vi "UHR-Fleezers Control (host) - 12.0(oscillate_test).vi"() -> ()   [LabVIEW 2014] (continued)
            n2102 = Wait (ms)(milliseconds to wait=u32 250) -> ()  [unwired: 1 out]
          }
          frame #5 {
            n2103 = case shown="\"1\"" "Remove Action Offset Dropdown" {
              tunnel: TRUE ("Value (Signaling)") -> [w3014 w3022 w3030]
              frame "1" {
                n2104 = flat-sequence {
                  tunnel: w3014 -> [w3021]
                  frame #0 {
                    n2105 = local read "factor"() -> (w3016:dbl)
                    n2106 = Greater Than 0?(x=w3016) -> (x > 0?=w3020:bool)
                    n2107 = Select(t=1.0, s=w3020, f=-1.0) -> (s? t:f=w3017:dbl)
                    n2108 = Multiply(x=w3017, y=w3016) -> (x*y=w3015:dbl)
                    n2109 = local write "factor"(w3015) -> ()
                  }
                  frame #1 {
                    n2110 = property on="Remove Offset to factor" class="Bool (strict)"("Val(Sgnl)"=w3021) -> ()  [unwired: 2 in, 2 out]
                  }
                }
              }
              frame "2" {
                n2111 = flat-sequence {
                  tunnel: w3022 -> [w3029]
                  frame #0 {
                    n2112 = local read "factor"() -> (w3023:dbl)
                    n2113 = Greater Than 0?(x=w3023) -> (x > 0?=w3028:bool)
                    n2114 = Select(t=-1.0, s=w3028, f=1.0) -> (s? t:f=w3026:dbl)
                    n2115 = Multiply(x=w3023, y=w3026) -> (x*y=w3025:dbl)
                    n2116 = local write "factor"(w3025) -> ()
                  }
                  frame #1 {
                    n2117 = property on="Remove Offset to factor" class="Bool (strict)"("Val(Sgnl)"=w3029) -> ()  [unwired: 2 in, 2 out]
                  }
                }
              }
              frame "0", Default {
                n2118 = property on="Remove Action Offset" class="Bool (strict)"("Val(Sgnl)"=w3030) -> ()  [unwired: 2 in, 2 out]
              }
            }
            n2119 = case shown="False" "Trap Trig Fl." {
              frame False {
                n2120 = case shown="True" "Green ON after FB ON?" {
                  selector: "Green ON after FB ON?" -> [_ w3032]
                  frame False {
                  }
                  frame True {
                    n2121 = property on="Green ON/Interlacing" class="Bool (strict)"("Val(Sgnl)"=w3032) -> ()  [unwired: 2 in, 2 out]
                  }
                }
              }
              frame True {
              }
            }
            n2122 = Wait (ms)(milliseconds to wait=u32 250) -> ()  [unwired: 1 out]
          }
          frame #6 {
            n2123 = property on="Start Saving" class="Bool (strict)"("Val(Sgnl)"=TRUE ("Value (Signaling)")) -> ()  [unwired: 2 in, 2 out]
            n2124 = Wait (ms)(milliseconds to wait=u32 5000) -> ()  [unwired: 1 out]
          }
          frame #7 {
            w3036 = TRUE ("Value (Signaling)")
            n2125 = property on="Rem fb disp offset" class="Bool (strict)"("Val(Sgnl)"=w3036) -> ()  [unwired: 2 in, 2 out]
            n2126 = property on="Remove Offset" class="Bool (strict)"("Val(Sgnl)"=w3036) -> ()  [unwired: 2 in, 2 out]
            n2127 = Wait (ms)(milliseconds to wait=u32 100) -> ()  [unwired: 1 out]
          }
          frame #8 {
            n2128 = case shown="True" w3039 {
              frame False {
              }
              frame True {
                n2129 = local write "Trap Trig. Fl."(TRUE ("Value (Signaling)")) -> ()
              }
            }
          }
          frame #9 {
            n2130 = local read "Tether"() -> (w3042:bool)
            n2131 = And(x="Start dipping after?", y=w3042) -> (x .and. y?=w3041:bool)
            n2132 = case shown="True" w3041 {
              frame False {
              }
              frame True {
                n2133 = flat-sequence {
                  frame #0 {
                    n2134 = Multiply(x="Delay before dipping (s)", y=1000.0) -> (x*y=w3045:dbl)
                    n2135 = Wait (ms)(milliseconds to wait=w3045) -> ()  [unwired: 1 out]
                  }
                  frame #1 {
                    n2136 = property on="Dip for Protein" class="Bool (strict)"("Val(Sgnl)"=TRUE ("Value (Signaling)")) -> ()  [unwired: 2 in, 2 out]
                    n2137 = local write "Scripts"(T35."Dipping") -> ()
                  }
                }
              }
            }
          }
        }
      }
      event "Rupture Script": Value Change {
        n2138 = event-data() -> ()  [unwired: 1 in, 5 out]
        n2139 = local write "Rupture Script"(FALSE ("Rupture Script")) -> ()
        n2140 = flat-sequence {
          frame #0 {
            w3051 = TRUE
            w3056 = FALSE
            # "Number 6 for now is the\nrupture-experiment\nparameters."
            n2141 = local read "Starting Trap D (MHz)"() -> (w3057:dbl)
            n2142 = local write "Restart DMA? (AOD)"(w3056) -> ()
            n2143 = Replace Array Subset(array=u32[] [0] ("Index Values"), new element=6, index=0) -> (w3052:u32[])
            n2144 = local write "Save scans"(w3056) -> ()
            n2145 = property on="Trap D (MHz)" class="DigNum (strict)"("Val(Sgnl)"=w3057) -> ()  [unwired: 2 in, 2 out]
            n2146 = property on="Saved AOD Raster Scan Parameter Sets" class="Arr (strict)"("Index Values"=w3052) -> ()  [unwired: 2 in, 2 out]
            n2147 = property on="Start Saving" class="Bool (strict)"("Val(Sgnl)"=w3051) -> ()  [unwired: 2 in, 2 out]
            n2148 = property on="Green ON/Interlacing" class="Bool (strict)"("Val(Sgnl)"=w3051) -> ()  [unwired: 2 in, 2 out]
          }
          frame #1 {
            n2149 = property on="Load parameters" class="Bool (strict)"("Val(Sgnl)"=TRUE ("Value (Signaling)")) -> ()  [unwired: 2 in, 2 out]
          }
        }
      }
      event "Fixed Traps Script": Value Change {
        n2150 = event-data() -> ()  [unwired: 1 in, 5 out]
        n2151 = local write "Fixed Traps Script"(FALSE ("Fixed Traps Data\nScript")) -> ()
        n2152 = flat-sequence {
          frame #0 {
            n2153 = case shown="True" "Green ON" {
              frame False {
              }
              frame True {
                n2154 = property on="Green ON/Interlacing" class="Bool (strict)"("Val(Sgnl)"=TRUE) -> ()  [unwired: 2 in, 2 out]
              }
            }
            n2155 = local write "Offset (nm)"(0.0 ("Offset (nm)")) -> ()
            n2156 = property on="Sample Channel\nFlow" class="Bool (strict)"("Val(Sgnl)"=FALSE ("Value (Signaling)")) -> ()  [unwired: 2 in, 2 out]
            n2157 = property on="Trap D (MHz)" class="DigNum (strict)"("Val(Sgnl)"="Fixed Traps Trap Delta (MHz)") -> ()  [unwired: 2 in, 2 out]
          }
          frame #1 {
            n2158 = Wait (ms)(milliseconds to wait=u32 1000) -> ()  [unwired: 1 out]
          }
          frame #2 {
            n2159 = local write "Start Saving"(TRUE ("Start Saving")) -> ()
          }
          frame #3 {
            n2160 = local read "Bead Sep. Int. Time (s)"() -> (w3067:dbl)
            n2161 = Multiply(x=w3067, y=1000.0) -> (x*y=w3069:dbl)
            n2162 = Wait (ms)(milliseconds to wait=w3069) -> ()  [unwired: 1 out]
          }
          frame #4 {
            n2163 = property on="Remove Offset" class="Bool (strict)"("Val(Sgnl)"=TRUE ("Value (Signaling)")) -> ()  [unwired: 2 in, 2 out]
          }
          frame #5 {
            n2164 = property on="Dip for Protein" class="Bool (strict)"("Val(Sgnl)"="Start dipping after?") -> ()  [unwired: 2 in, 2 out]
          }
        }
      }
      event "Got DNA bead": Value Change {
        n2165 = event-data() -> ()  [unwired: 1 in, 5 out]
        n2166 = flat-sequence {
          frame #0 {
            w3073 = FALSE ("Key Focus")
            n2167 = local read "Daq spot flow on"() -> (w3074:bool)
            n2168 = case shown="True" w3074 {
              frame False {
              }
              frame True {
                n2169 = property on="Sample Channel\nFlow" class="Bool (strict)"("Val(Sgnl)"=TRUE ("Value (Signaling)")) -> ()  [unwired: 2 in, 2 out]
              }
            }
            n2170 = local write "Got DNA bead"(w3073) -> ()
            n2171 = property on="Got DNA bead" class="Bool (strict)"("Key Focus"=w3073) -> ()  [unwired: 2 in, 2 out]
          }
          frame #1 {
            n2172 = property on="Inject Pump 1" class="Bool (strict)"("Val(Sgnl)"=FALSE ("Value (Signaling)")) -> ()  [unwired: 2 in, 2 out]
          }
          frame #2 {
            n2173 = property on="Cal/Data Acq. Spot" class="Bool (strict)"("Val(Sgnl)"=TRUE ("Value (Signaling)")) -> ()  [unwired: 2 in, 2 out]
          }
        }
      }
      event "Take Stepping Data": Value Change {
        n2174 = event-data() -> ()  [unwired: 1 in, 5 out]
        n2175 = local read "Save ave N"() -> (w3086:dbl)
        n2176 = flat-sequence {
          tunnel: w3086 -> [w3088]
          tunnel: [w3088] -> w3081
          tunnel: [w3090] -> w3082
          tunnel: w3081 -> [w3090]
          tunnel: [w3092] -> w3083
          tunnel: w3082 -> [w3092]
          tunnel: [w3095] -> w3084
          tunnel: w3083 -> [w3095]
          tunnel: [w3097] -> w3085
          tunnel: w3084 -> [w3097]
          tunnel: [w3099] -> w3079
          tunnel: w3085 -> [w3099]
          tunnel: w3079 -> [w3102]
          tunnel: [w3102] -> w3078
          tunnel: w3078 -> [w3103]
          tunnel: [w3103] -> w3080
          tunnel: w3080 -> [w3109]
          frame #0 {
            n2177 = property on="Save ave N" class="DigNum (strict)"("Val(Sgnl)"="Save ave factor") -> ()  [unwired: 2 in, 2 out]
          }
          frame #1 {
            n2178 = Wait (ms)(milliseconds to wait=u32 100) -> ()  [unwired: 1 out]
          }
          frame #2 {
            n2179 = local read "Offset 2 Start (MHz)"() -> (w3094:dbl)
            n2180 = property on="Saved AOD Raster Scan Parameter Sets" class="Arr (strict)"("Index Values"=u32[] [2]) -> ()  [unwired: 2 in, 2 out]
            n2181 = property on="Trap D (MHz)" class="DigNum (strict)"("Val(Sgnl)"=w3094) -> ()  [unwired: 2 in, 2 out]
          }
          frame #3 {
            n2182 = property on="Load parameters" class="Bool (strict)"("Val(Sgnl)"=TRUE ("Value (Signaling)")) -> ()  [unwired: 2 in, 2 out]
          }
          frame #4 {
            n2183 = Wait (ms)(milliseconds to wait=u32 100) -> ()  [unwired: 1 out]
          }
          frame #5 {
            n2184 = property on="Trap Raster Scan" class="Bool (strict)"("Val(Sgnl)"=TRUE ("Value (Signaling)")) -> ()  [unwired: 2 in, 2 out]
          }
          frame #6 {
            n2185 = Wait (ms)(milliseconds to wait=u32 1000) -> ()  [unwired: 1 out]
          }
          frame #7 {
            n2186 = while {
              stop <- w3106 stop-if-true
              n2187 = local read "Raster Scanning..."() -> (w3108:bool)
              n2188 = local read "Saving..."() -> (w3107:bool)
              n2189 = Not(x=w3107) -> (.not. x?=w3104:bool)
              n2190 = Not(x=w3108) -> (.not. x?=w3105:bool)
              n2191 = And(x=w3105, y=w3104) -> (x .and. y?=w3106:bool)
            }
          }
          frame #8 {
            n2192 = property on="Save ave N" class="DigNum (strict)"("Val(Sgnl)"=w3109) -> ()  [unwired: 2 in, 2 out]
          }
        }
      }
      event "Step Size (nm)": Value Change {
        n2193 = event-data() -> ()  [unwired: 1 in, 5 out]
        n2194 = flat-sequence {
          frame #0 {
            n2195 = property on="Saved AOD Raster Scan Parameter Sets" class="Arr (strict)"("Index Values"=u32[] [1]) -> ()  [unwired: 2 in, 2 out]
          }
          frame #1 {
            n2196 = Multiply(x="N Steps", y="Step Size (nm)") -> (x*y=w3111:dbl)
            n2197 = property on="Scan Speed AOD (nm/s) 2" class="DigNum (strict)"("Value"="Step Size (nm)") -> ()  [unwired: 2 in, 2 out]
            n2198 = property on="Step Size AOD (nm) 2" class="DigNum (strict)"("Value"="Step Size (nm)") -> ()  [unwired: 2 in, 2 out]
            n2199 = property on="Scan Range AOD (nm) 2" class="DigNum (strict)"("Value"=w3111) -> ()  [unwired: 2 in, 2 out]
          }
        }
      }
      event "Take Detection Laser\nImage": Value Change {
        n2200 = event-data() -> ()  [unwired: 1 in, 5 out]
        n2201 = flat-sequence {
          tunnel: [w3139] -> w3129
          tunnel: [w3138] -> w3122
          tunnel: [w3137] -> w3114
          tunnel: [w3142] -> w3130
          tunnel: w3129 -> [w3142]
          tunnel: [w3141] -> w3123
          tunnel: w3122 -> [w3141]
          tunnel: [w3140] -> w3115
          tunnel: w3114 -> [w3140]
          tunnel: [w3146] -> w3131
          tunnel: w3130 -> [w3146]
          tunnel: [w3145] -> w3124
          tunnel: w3123 -> [w3145]
          tunnel: [w3144] -> w3116
          tunnel: w3115 -> [w3144]
          tunnel: [w3152] -> w3132
          tunnel: w3131 -> [w3152]
          tunnel: [w3151] -> w3125
          tunnel: w3124 -> [w3151]
          tunnel: [w3150] -> w3117
          tunnel: w3116 -> [w3150]
          tunnel: [w3156] -> w3133
          tunnel: w3132 -> [w3156]
          tunnel: [w3155] -> w3126
          tunnel: w3125 -> [w3155]
          tunnel: [w3154] -> w3118
          tunnel: w3117 -> [w3154]
          tunnel: [w3160] -> w3134
          tunnel: w3133 -> [w3160]
          tunnel: [w3159] -> w3127
          tunnel: w3126 -> [w3159]
          tunnel: [w3158] -> w3119
          tunnel: w3118 -> [w3158]
          tunnel: [w3164] -> w3135
          tunnel: w3134 -> [w3164]
          tunnel: [w3163] -> w3128
          tunnel: w3127 -> [w3163]
          tunnel: [w3162] -> w3120
          tunnel: w3119 -> [w3162]
          tunnel: w3135 -> [w3170]
          tunnel: w3128 -> [w3169]
          tunnel: [w3167] -> w3121
          tunnel: w3120 -> [w3167]
          tunnel: w3121 -> [w3171]
          frame #0 {
            n2202 = local read "Laser interlacing mode (all lasers)"() -> (w3138:enum32{"Laser ON", "Laser OFF", "Interlace"})
            n2203 = local read "Green ON/Interlacing"() -> (w3139:bool)
            n2204 = local read "Green FB On/Off"() -> (w3137:bool)
          }
          frame #1 {
            n2205 = property on="Green FB On/Off" class="Bool (strict)"("Val(Sgnl)"=FALSE ("Value (Signaling)")) -> ()  [unwired: 2 in, 2 out]
          }
          frame #2 {
            n2206 = property on="Green ON/Interlacing" class="Bool (strict)"("Val(Sgnl)"=TRUE ("Value (Signaling)")) -> ()  [unwired: 2 in, 2 out]
            n2207 = property on="Flip Green Filter" class="Bool (strict)"("Val(Sgnl)"=TRUE ("Value (Signaling)")) -> ()  [unwired: 2 in, 2 out]
            n2208 = property on="Laser interlacing mode (all lasers)" class="RadioBtnsControl (strict)"("Val(Sgnl)"=enum32{"Laser ON", "Laser OFF", "Interlace"}."Laser ON" ("Value (Signaling)")) -> ()  [unwired: 2 in, 2 out]
          }
          frame #3 {
            n2209 = Wait (ms)(milliseconds to wait=u32 500) -> ()  [unwired: 1 out]
          }
          frame #4 {
            n2210 = property on="Confocal\nImage" class="Bool (strict)"("Val(Sgnl)"=TRUE ("Value (Signaling)")) -> ()  [unwired: 2 in, 2 out]
          }
          frame #5 {
            n2211 = Wait (ms)(milliseconds to wait=u32 2000) -> ()  [unwired: 1 out]
          }
          frame #6 {
            n2212 = while {
              stop <- w3165 stop-if-true
              n2213 = local read "Saving..."() -> (w3166:bool)
              n2214 = Not(x=w3166) -> (.not. x?=w3165:bool)
            }
          }
          frame #7 {
            n2215 = property on="Flip Green Filter" class="Bool (strict)"("Val(Sgnl)"=TRUE ("Value (Signaling)")) -> ()  [unwired: 2 in, 2 out]
            n2216 = property on="Green ON/Interlacing" class="Bool (strict)"("Val(Sgnl)"=w3170) -> ()  [unwired: 2 in, 2 out]
            n2217 = property on="Laser interlacing mode (all lasers)" class="RadioBtnsControl (strict)"("Val(Sgnl)"=w3169) -> ()  [unwired: 2 in, 2 out]
          }
          frame #8 {
            n2218 = property on="Green FB On/Off" class="Bool (strict)"("Val(Sgnl)"=w3171) -> ()  [unwired: 2 in, 2 out]
          }
        }
      }
      event "Stop All": Value Change {
        n2219 = event-data() -> ()  [unwired: 1 in, 5 out]
        n2220 = local read "Stop All"() -> (w3172:bool)
      }
    }
    n2221 = node-c288() -> ()  [unwired: 1 in, 1 out]
  }
  n2222 = node-c288() -> (w139:T26)  [unwired: 4 out]
  n2223 = timed-loop "Mouse control: trap position (AOM deflection), set confocal spot from image" {
    tunnel: [w3174] -> w224
    tunnel: w51 -> [w3173]
    timing: w139 -> [_]
    timing-out: [_] -> w138
    stop <- w3174 stop-if-true
    n2224 = node-c288() -> ()  [unwired: 2 out]
    n2225 = event shown="[0] \"Pane\": Mouse Down" {
      selector: _ -> [_ _]
      dyn-events: _ -> [_ _]
      timeout: _ -> [_ _]
      tunnel: w3173 -> [w3177 _]
      event Mouse Down {
        n2226 = event-data() -> ("Time"=w3179:u32, "Coords"=w3178:T7, "Button"=w3180:u16)  [unwired: 6 out]
        n2227 = case shown="1" w3180 {
          tunnel: w3179 -> [_ _ w3319]
          tunnel: w3178 -> [_ w3185 w3317]
          tunnel: w3177 -> [_ _ w3315]
          frame 0, Default {
          }
          frame 1 {
            n2228 = property on="APD 2" class="ImageControl"() -> ("Displayed Image Position"=w3199:cluster{"Left":i32, "Top":i32})  [unwired: 2 in, 2 out]
            n2229 = control-ref of="Primary Video Display"() -> (w3192:refnum<vi>)
            n2230 = property on="APD 1" class="ImageControl"() -> ("Displayed Image Position"=w3228:cluster{"Left":i32, "Top":i32})  [unwired: 2 in, 2 out]
            n2231 = property on="Detection Laser X" class="ImageControl"() -> ("Displayed Image Position"=w3225:cluster{"Left":i32, "Top":i32})  [unwired: 2 in, 2 out]
            n2232 = property on="Detection Laser Y" class="ImageControl"() -> ("Displayed Image Position"=w3224:cluster{"Left":i32, "Top":i32})  [unwired: 2 in, 2 out]
            n2233 = property on="APD 2" class="ImageControl"() -> ("Displayed Image Size"=w3198:cluster{"Width":u32, "Height":u32})  [unwired: 2 in, 2 out]
            n2234 = property on="APD 1" class="ImageControl"() -> ("Displayed Image Size"=w3226:cluster{"Width":u32, "Height":u32})  [unwired: 2 in, 2 out]
            n2235 = property on="Detection Laser X" class="ImageControl"() -> ("Displayed Image Size"=w3227:cluster{"Width":u32, "Height":u32})  [unwired: 2 in, 2 out]
            n2236 = property on="Detection Laser Y" class="ImageControl"() -> ("Displayed Image Size"=w3223:cluster{"Width":u32, "Height":u32})  [unwired: 2 in, 2 out]
            n2237 = property class="ImageControl"(reference=w3192) -> ("Displayed Image Position"=w3190:cluster{"Left":i32, "Top":i32})  [unwired: 1 in, 2 out]
            n2238 = property class="ImageControl"(reference=w3192) -> ("Displayed Image Size"=w3191:cluster{"Width":u32, "Height":u32})  [unwired: 1 in, 2 out]
            n2239 = Unbundle By Name(w3198) -> ("Width"=w3195:u32, "Height"=w3194:u32)
            n2240 = Unbundle By Name(w3199) -> ("Left"=w3197:i32, "Top"=w3196:i32)
            n2241 = Unbundle By Name(w3226) -> ("Width"=w3220:u32, "Height"=w3219:u32)
            n2242 = Unbundle By Name(w3227) -> ("Width"=w3216:u32, "Height"=w3215:u32)
            n2243 = Unbundle By Name(w3223) -> ("Width"=w3212:u32, "Height"=w3211:u32)
            n2244 = Unbundle By Name(w3228) -> ("Left"=w3222:i32, "Top"=w3221:i32)
            n2245 = Unbundle By Name(w3225) -> ("Left"=w3218:i32, "Top"=w3217:i32)
            n2246 = Unbundle By Name(w3224) -> ("Left"=w3214:i32, "Top"=w3213:i32)
            n2247 = Bundle("Left"=w3197, "Top"=w3196, "Width"=w3195, "Height"=w3194) -> (w3193:T36)  [unwired: 1 in]
            n2248 = Bundle("Left"=w3222, "Top"=w3221, "Width"=w3220, "Height"=w3219) -> (w3210:T36)  [unwired: 1 in]
            n2249 = Bundle("Left"=w3218, "Top"=w3217, "Width"=w3216, "Height"=w3215) -> (w3209:T36)  [unwired: 1 in]
            n2250 = Bundle("Left"=w3214, "Top"=w3213, "Width"=w3212, "Height"=w3211) -> (w3208:T36)  [unwired: 1 in]
            n2251 = Unbundle By Name(w3191) -> ("Width"=w3187:u32, "Height"=w3186:u32)
            n2252 = Unbundle By Name(w3190) -> ("Left"=w3189:i32, "Top"=w3188:i32)
            n2253 = Build Cluster Array(w3193, w3210, w3209, w3208) -> (w3207:T37)
            n2254 = Bundle("Left"=w3189, "Top"=w3188, "Width"=w3187, "Height"=w3186) -> (w3182:T36)  [unwired: 1 in]
            n2255 = for {
              tunnel: w3185 -> [w3261]
              tunnel: w3207 -> [w3262] mode=indexing
              shift-right: [w3259] -> w3205
              shift-left: TRUE -> [w3260]
              shift-right: [w3258] -> w3203
              shift-left: _ -> [w3254]
              shift-right: [w3257] -> w3202
              shift-left: _ -> [w3253]
              shift-right: [w3256] -> w3201
              shift-left: _ -> [w3252]
              shift-right: [w3255] -> w3200
              shift-left: _ -> [w3251]
              n2256 = case shown="True" w3260 {
                selector: w3260 -> [w3267 _]
                tunnel: w3262 -> [_ w3276]
                tunnel: w3261 -> [_ w3274]
                tunnel: [w3267 w3272] -> w3259
                tunnel: [w3266 w3271] -> w3258
                tunnel: [w3265 w3270] -> w3257
                tunnel: [w3264 w3269] -> w3256
                tunnel: [w3263 w3268] -> w3255
                tunnel: w3254 -> [w3266 _]
                tunnel: w3253 -> [w3265 _]
                tunnel: w3252 -> [w3264 _]
                tunnel: w3251 -> [w3263 _]
                frame False {
                }
                frame True {
                  n2257 = Unbundle(w3276) -> (w3275:T36)
                  n2258 = call "isclickinwindow.vi"("Image Param"=w3275, "Point32"=w3274) -> ("4 Y"=w3268:i32, "3 Height"=w3269:i32, "2 X"=w3270:i32, "1 Width"=w3271:i32, "In image?"=w3273:bool)  [unwired: 1 in]
                  n2259 = Not(x=w3273) -> (.not. x?=w3272:bool)
                }
              }
            }
            n2260 = call "isclickinwindow.vi"("Image Param"=w3182, "Point32"=w3185) -> ("4 Y"=w3183:i32, "2 X"=w3184:i32, "In image?"=w3181:bool)  [unwired: 1 in, 2 out]
            n2261 = case shown="True" w3181 {
              tunnel: w3184 -> [_ w3232]
              tunnel: w3183 -> [_ w3235]
              frame False {
              }
              frame True {
                w3244 = 2
                n2262 = Subtract(x=480, y=w3235) -> (x-y=w3234:i32)
                n2263 = Unbundle("Target size") -> ("Width"=w3245:dbl, "Height"=w3243:dbl)
                n2264 = Subtract(x=w3232, y=2) -> (x-y=w3231:i32)
                n2265 = Divide(x=w3243, y=w3244) -> (x/y=w3241:dbl)
                n2266 = Divide(x=w3245, y=w3244) -> (x/y=w3242:dbl)
                n2267 = Subtract(x=w3231, y=w3242) -> (x-y=w3240:dbl)
                n2268 = Add(x=w3231, y=w3242) -> (x+y=w3238:dbl)
                n2269 = Subtract(x=w3234, y=w3241) -> (x-y=w3239:dbl)
                n2270 = Add(x=w3234, y=w3241) -> (x+y=w3237:dbl)
                n2271 = Bundle(w3231, w3234) -> (w3247:cluster{i32, i32})  [unwired: 1 in]
                n2272 = Bundle(w3240, w3239, w3238, w3237) -> (w3229:cluster{dbl, dbl, dbl, dbl})  [unwired: 1 in]
                n2273 = case shown="True" "Set target" {
                  tunnel: w3247 -> [_ w3250]
                  tunnel: w3229 -> [_ w3248]
                  frame False {
                  }
                  frame True {
                    n2274 = local write "Target coordinates"(w3248) -> ()
                    n2275 = local write "Set target"(FALSE ("Set target")) -> ()
                    "Video coordinates" <- w3250
                  }
                }
              }
            }
            n2276 = Not(x=w3205) -> (.not. x?=w3204:bool)
            n2277 = case shown="True" w3204 {
              tunnel: w3202 -> [_ w3290]
              tunnel: w3200 -> [_ w3289]
              tunnel: w3203 -> [_ w3288]
              tunnel: w3201 -> [_ w3287]
              frame False {
              }
              frame True {
                w3277 = FALSE ("Get Point")
                n2278 = local read "Scan lines (y)"() -> (w3292:u64)
                n2279 = disable-structure shown="Disabled" {
                  frame Disabled {
                  }
                  frame Enabled {
                  }
                }
                n2280 = local read "Actual MCL Inc (V)"() -> (w3286:dbl)
                n2281 = local read "Scan steps (MCL)"() -> (w3291:u64)
                n2282 = Divide "Y Pix/step"(x=w3287, y=w3292) -> (x/y=w3299:dbl)
                n2283 = Divide "Y V/pix"(x=w3286, y=w3299) -> (x/y=w3298:dbl)
                n2284 = Divide "Y half step offset"(x=w3286, y=2.0) -> (x/y=w3300:dbl)
                n2285 = Divide "X pix/step"(x=w3288, y=w3291) -> (x/y=w3297:dbl)
                n2286 = Negate(x=w3300) -> (-x=w3301:dbl)
                n2287 = local read "Initial Y"() -> (w3307:dbl)
                n2288 = Multiply(x=w3289, y=w3298) -> (x*y=w3308:dbl)
                n2289 = Divide "X half step offset"(x=w3286, y=2.0) -> (x/y=w3294:dbl)
                n2290 = Divide "X V/pix"(x=w3286, y=w3297) -> (x/y=w3296:dbl)
                n2291 = Multiply(x=w3286, y=w3291) -> (x*y=w3303:dbl)
                n2292 = Compound Arithmetic op=ADD(w3301, w3308, w3307) -> (w3278:dbl)
                "Pointer Y (V)" <- w3278
                n2293 = Multiply(x=w3296, y=w3290) -> (x*y=w3305:dbl)
                n2294 = Negate(x=w3294) -> (-x=w3293:dbl)
                n2295 = local read "Initial X"() -> (w3306:dbl)
                n2296 = Negate(x=w3305) -> (-x=w3304:dbl)
                n2297 = Compound Arithmetic op=ADD(w3293, w3303, w3306, w3304) -> (w3279:dbl)
                "Pointer X (V)" <- w3279
                n2298 = case shown="True" "Set High F Confocal Spot (X-Y)" {
                  tunnel: w3279 -> [_ w3309]
                  tunnel: w3278 -> [_ w3310]
                  frame False {
                  }
                  frame True {
                    "Confocal Y 2 (V)" <- w3310
                    "Confocal X 2 (V)" <- w3309
                  }
                }
                n2299 = Or(x="Set X Only", y="Set Confocal Spot (X-Y)") -> (x .or. y?=w3282:bool)
                n2300 = Or(x="Set Confocal Spot (X-Y)", y="Set Y Only") -> (x .or. y?=w3281:bool)
                n2301 = case shown="True" w3282 {
                  tunnel: w3279 -> [_ w3311]
                  frame False {
                  }
                  frame True {
                    n2302 = property on="AO2" class="Slide (strict)"("Val(Sgnl)"=w3311) -> ()  [unwired: 2 in, 2 out]
                    "Confocal X 1 (V)" <- w3311
                  }
                }
                n2303 = case shown="True" w3281 {
                  tunnel: w3278 -> [_ w3312]
                  frame False {
                  }
                  frame True {
                    n2304 = property on="AO1" class="Slide (strict)"("Val(Sgnl)"=w3312) -> ()  [unwired: 2 in, 2 out]
                    "Confocal Y 1 (V)" <- w3312
                  }
                }
                n2305 = local write "Set High F Confocal Spot (X-Y)"(w3277) -> ()
                n2306 = local write "Set Confocal Spot (X-Y)"(w3277) -> ()
                n2307 = local write "Set X Only"(w3277) -> ()
                n2308 = local write "Set Y Only"(w3277) -> ()
              }
            }
          }
          frame 3 {
            n2309 = local read "BD 2 Frequency 1 (MHz)"() -> (w3313:dbl)
            n2310 = local read "BD 1 Frequency 1 (MHz)"() -> (w3314:dbl)
            n2311 = local write "Manipulating Trap"(TRUE ("Manipulating Trap")) -> ()
            n2312 = local write "Coords"(T7 {"Horizontal"=0, "Vertical"=0} ("Coords")) -> ()
            n2313 = while {
              tunnel: w3319 -> [w3324]
              tunnel: w3317 -> [w3323]
              tunnel: w3315 -> [w3322]
              tunnel: w3314 -> [w3321]
              tunnel: w3313 -> [w3320]
              stop <- w3325 stop-if-true
              n2314 = event shown="[0] \"Pane\": Mouse Move" {
                selector: _ -> [_ _]
                dyn-events: _ -> [_ _]
                timeout: _ -> [_ _]
                tunnel: ["Force Manip Abort" w3389] -> w3325
                tunnel: w3324 -> [w3332 _]
                tunnel: w3323 -> [w3330 _]
                tunnel: w3322 -> [w3329 _]
                tunnel: w3321 -> [w3328 _]
                tunnel: w3320 -> [w3327 _]
                event Mouse Move {
                  n2315 = event-data() -> ("Time"=w3333:u32, "Coords"=w3334:T7)  [unwired: 3 out]
                  n2316 = Less?(x=w3333, y=w3332) -> (x < y?=w3331:bool)
                  n2317 = case "Makes sure old motion events prior to mouse click aren't used" shown="False" w3331 {
                    tunnel: w3334 -> [w3376 _]
                    tunnel: w3330 -> [w3377 _]
                    tunnel: w3329 -> [w3354 _]
                    tunnel: w3328 -> [w3350 _]
                    tunnel: w3327 -> [w3349 _]
                    frame False {
                      n2318 = Subtract(x=w3376, y=w3377) -> (x-y=w3375:T7)
                      "Coords" <- w3375
                      n2319 = local read "Y RF Frequency Limits (MHz)"() -> (w3335:T17)
                      n2320 = To Double Precision Float(number=w3375) -> (double precision float=w3374:cluster{"Horizontal":dbl, "Vertical":dbl})
                      n2321 = Multiply(x=cluster{"Horizontal":dbl, "Vertical":dbl} {"Horizontal"=-1.0, "Vertical"=1.0}, y="Manipulation Scaling") -> (x*y=w3370:cluster{"Horizontal":dbl, "Vertical":dbl})
                      n2322 = local read "X RF Frequency Limits (MHz)"() -> (w3336:T17)
                      n2323 = Multiply(x=w3374, y=w3370) -> (x*y=w3372:cluster{"Horizontal":dbl, "Vertical":dbl})
                      n2324 = Unbundle By Name(w3372) -> ("Horizontal"=w3367:dbl, "Vertical"=w3371:dbl)
                      n2325 = Unbundle By Name(w3335) -> ("Maximum"=w3338:dbl, "Minimum"=w3337:dbl)
                      n2326 = Boolean To (0,1)(Boolean="Manip. X?") -> (0, 1=w3365:i16)
                      n2327 = Boolean To (0,1)(Boolean="Manip. Y?") -> (0, 1=w3362:i16)
                      n2328 = local read "BD 1 Frequency 2 (MHz)"() -> (w3352:dbl)
                      n2329 = Multiply(x=w3371, y=w3362) -> (x*y=w3364:dbl)
                      n2330 = Multiply(x=w3365, y=w3367) -> (x*y=w3368:dbl)
                      n2331 = local read "BD 2 Frequency 2 (MHz)"() -> (w3351:dbl)
                      n2332 = Unbundle By Name(w3336) -> ("Maximum"=w3340:dbl, "Minimum"=w3339:dbl)
                      n2333 = Add(x=w3349, y=w3364) -> (x+y=w3342:dbl)
                      n2334 = Add(x=w3350, y=w3368) -> (x+y=w3344:dbl)
                      n2335 = In Range and Coerce(upper limit=w3340, x=w3344, lower limit=w3339) -> (coerced(x)=w3343:dbl)  [unwired: 1 out]
                      n2336 = In Range and Coerce(upper limit=w3338, x=w3342, lower limit=w3337) -> (coerced(x)=w3341:dbl)  [unwired: 1 out]
                      n2337 = Subtract(x=w3343, y=w3352) -> (x-y=w3361:dbl)
                      n2338 = Subtract(x=w3341, y=w3351) -> (x-y=w3360:dbl)
                      n2339 = Square(x=w3361) -> (x^2=w3359:dbl)
                      n2340 = Square(x=w3360) -> (x^2=w3358:dbl)
                      n2341 = Add(x=w3359, y=w3358) -> (x+y=w3357:dbl)
                      n2342 = Square Root(x=w3357) -> (sqrt(x)=w3353:dbl)
                      n2343 = In Range and Coerce(upper limit="Limit Max (MHz)", x=w3353, lower limit="Limit Min (MHz)") -> (In Range?=w3346:bool)  [unwired: 1 out]
                      n2344 = Not(x="Limits Enable") -> (.not. x?=w3345:bool)
                      n2345 = Or(x=w3346, y=w3345) -> (x .or. y?=w3347:bool)
                      n2346 = case shown="True" w3347 {
                        tunnel: w3354 -> [_ w3387]
                        tunnel: w3353 -> [_ w3378]
                        tunnel: w3343 -> [_ w3385]
                        tunnel: w3352 -> [_ w3384]
                        tunnel: w3341 -> [_ w3383]
                        tunnel: w3351 -> [_ w3382]
                        tunnel: w3336 -> [_ w3380]
                        tunnel: w3335 -> [_ w3379]
                        frame False {
                        }
                        frame True {
                          n2347 = local read "BD 1 Frequency 3 (MHz)"() -> (w3386:dbl)
                          n2348 = local read "BD 2 Frequency 3 (MHz)"() -> (w3381:dbl)
                          n2349 = local write "Trap D (MHz)"(w3378) -> ()
                          n2350 = call "set RF board frequency - interlace.vi"("Board 2 Frequency Limits"=w3379, "Board 1 Frequency Limits"=w3380, "FPGA VI Reference In"=w3387, "Board 2 Frequency 3 (MHz)"=w3381, "Board 1 Frequency 3 (MHz)"=w3386, "Board 2 Frequency 2 (MHz)"=w3382, "Board 2 Frequency 1 (MHz)"=w3383, "Board 1 Frequency 2 (MHz)"=w3384, "Board 1 Frequency 1  (MHz)"=w3385) -> ()  [unwired: 1 in, 2 out]
                          n2351 = local write "BD 2 Frequency 1 (MHz)"(w3383) -> ()
                          n2352 = local write "BD 1 Frequency 1 (MHz)"(w3385) -> ()
                        }
                      }
                    }
                    frame True {
                    }
                  }
                }
                event Mouse Up {
                  n2353 = event-data() -> ("Button"=w3388:u16)  [unwired: 8 out]
                  n2354 = case shown="3" w3388 {
                    tunnel: [FALSE TRUE] -> w3389
                    frame 0, Default {
                    }
                    frame 3 {
                      n2355 = local read "Trap D (MHz)"() -> (w3391:dbl)
                      n2356 = property on="Initial D (MHz)" class="DigNum (strict)"("Val(Sgnl)"=w3391) -> ()  [unwired: 2 in, 2 out]
                      n2357 = local write "Manipulating Trap"(FALSE ("Manipulating Trap")) -> ()
                    }
                  }
                }
              }
            }
          }
        }
      }
      event Mouse Move {
        n2358 = event-data() -> ()  [unwired: 6 out]
      }
    }
    n2359 = local read "Stop All"() -> (w3174:bool)
    n2360 = node-c288() -> ()  [unwired: 2 out]
  }
  n2361 = node-c288(w136) -> ()  [unwired: 1 out]
  n2362 = node-c288(w138) -> ()  [unwired: 1 out]
  n2363 = node-c288(w125) -> ()  [unwired: 1 out]
  n2364 = flat-sequence "Video" {
    tunnel: [w3402] -> w127
    tunnel: w127 -> [w3443]
    frame #0 {
      n2365 = while {
        stop <- w3395 continue-if-true
        n2366 = call "Close Video Capture.vi"() -> ("error code OUT"=w3397:i32)
        n2367 = Equal?(x=w3397, y=0) -> (x = y?=w3395:bool)
      }
      n2368 = local write "Stop All"(FALSE ("Stop All")) -> ()
    }
    frame #1 {
      n2369 = call "DMR_Init.vi"() -> ()  [unwired: 3 out]
    }
    frame #2 {
      # "Setting the destination format to Mono8 makes sure that the image can be displayed in the intensity plot."
      n2370 = call "DMR_GetDevice.vi"("search string IN"="DE019116701") -> ("device handle OUT"=w3420:i32)  [unwired: 4 in, 2 out]
      n2371 = call "DMR_OpenDevice.vi"("device handle IN"=w3420) -> ("driver handle OUT"=w3403:i32)  [unwired: 4 out]
      n2372 = call "DMR_FindList.vi"("flags IN"=u32 0 ("flags"), "list name IN"="" ("String"), "list type IN"=T38."camera descriptions", "driver handle IN"=w3403) -> ("list handle OUT"=w3406:i32)  [unwired: 2 out]
      n2373 = call "DMR_FindList.vi"("flags IN"=u32 0 ("flags"), "list name IN"="Base", "list type IN"=T38."setting", "driver handle IN"=w3403) -> ("list handle OUT"=w3404:i32)  [unwired: 2 out]
      n2374 = call "OBJ_GetHandle.vi"("object name IN"="VideoStandard", "list handle IN"=w3406) -> ("object handle OUT"=w3400:i32)  [unwired: 3 out]
      n2375 = call "OBJ_GetHandle.vi"("object name IN"="PixelFormat", "list handle IN"=w3404) -> ("object handle OUT"=w3414:i32)  [unwired: 3 out]
      n2376 = call "OBJ_SetS.vi"("value index IN"=0, "value IN"="NTSC M", "object handle IN"=w3400) -> ()  [unwired: 2 out]
      n2377 = call "OBJ_SetS.vi"("value index IN"=0, "value IN"="Mono8" ("value"), "object handle IN"=w3414) -> ()  [unwired: 2 out]
      n2378 = call "OBJ_GetHandle.vi"("object name IN"="VideoChannel", "list handle IN"=w3404) -> ("object handle OUT"=w3410:i32)  [unwired: 3 out]
      n2379 = while {
        tunnel: [w3425] -> w3402
        tunnel: w3403 -> [w3422]
        stop <- w3423 continue-if-true
        n2380 = call "DMR_ImageRequestSingle.vi"("request control IN"=0, "driver handle IN"=w3422) -> ("error code OUT"=w3424:i32, "driver handle OUT"=w3425:i32)  [unwired: 2 out]
        n2381 = Equal To 0?(x=w3424) -> (x = 0?=w3423:bool)
      }
      n2382 = call "OBJ_SetI.vi"("value index IN"=0, "value IN"=3 ("Video channel"), "object handle IN"=w3410) -> ()  [unwired: 2 out]
    }
    frame #3 {
      w3431 = T20 0 items=["Grayscale (U8)", "Grayscale (I16)", "Grayscale (SGL)", "Complex (CSG)", "RGB (U32)", "HSL (U32)", "RGB (U64)"] ("Image Type")
      w3439 = T20 0 items=["Grayscale (U8)", "Grayscale (I16)", "Grayscale (SGL)", "Complex (CSG)", "RGB (U32)", "HSL (U32)", "RGB (U64)"] ("Image Type")
      n2383 = for "Create Greyscale map" {
        N: 256 -> [_]
        tunnel: [w3445] -> w3428 mode=indexing
        workers-P: _ -> [_]
        i -> [w3448]
        n2384 = To Unsigned Byte Integer(number=w3448) -> (unsigned 8bit integer=w3444:u8)
        n2385 = Join Numbers(hi=w3444, lo=w3444) -> ((hi.lo)=w3447:u16)
        n2386 = Join Numbers(hi=w3444, lo=w3444) -> ((hi.lo)=w3446:u16)
        n2387 = Join Numbers(hi=w3447, lo=w3446) -> ((hi.lo)=w3445:u32)
      }
      n2388 = call "IMAQ Create"("Image Name"="Scaled video", "Image Type"=w3431) -> ("New Image"=w3430:T2)  [unwired: 2 in, 2 out]
      n2389 = call "IMAQ Create"("Image Name"="Main video", "Image Type"=w3439) -> ("New Image"=w3440:T2)  [unwired: 2 in, 2 out]
      n2390 = node-c288(0 ("Processor")) -> (w3438:T26)  [unwired: 3 out]
      n2391 = Initialize Array(u32 0 ("Window Number (0...15)"), 480 ("dimension size"), 640 ("dimension size")) -> (w3433:u32[][])
      n2392 = timed-loop {
        tunnel: w3443 -> [w3465]
        tunnel: [w3464] -> w3442
        tunnel: w3440 -> [w3463]
        timing: w3438 -> [_]
        timing-out: [_] -> w3437
        tunnel: w3433 -> [w3452]
        tunnel: w3430 -> [w3450]
        tunnel: w3428 -> [w3449]
        stop <- w3451 stop-if-true
        # "This block performs the \nactual image capture."
        n2393 = node-c288() -> ()  [unwired: 2 out]
        n2394 = local read "Stop All"() -> (w3451:bool)
        n2395 = Reciprocal(x="Video Capture Rate (Hz)") -> (1/x=w3455:dbl)
        n2396 = Multiply(x=w3455, y=1000.0) -> (x*y=w3453:dbl)
        n2397 = call "DMR_ImageRequestWaitFor.vi"("queue number IN"=0, "timeout(ms) IN"=500, "driver handle IN"=w3465) -> ("error code OUT"=w3469:i32, "request number OUT"=w3466:i32, "driver handle OUT"=w3467:i32)
        n2398 = feedback #1(T39 refnum ("Avi Refnum")) -> (w3457:T39)
        n2399 = case shown="True" "New Video File" {
          tunnel: [T39 refnum ("Avi Refnum") w3486] -> w3459
          tunnel: [FALSE TRUE] -> w3460
          tunnel: w3457 -> [_ w3482]
          frame False {
          }
          frame True {
            n2400 = call "Create new save file.vi"("Ext"=".avi" ("string"), "Index In"="Video Index") -> ("Path Out"=w3478:path, "Index Out"=w3479:dbl)  [unwired: 1 in]
            "Path Out" <- w3478
            n2401 = Not Equal?(x=w3482, y=T39 refnum ("Avi Refnum")) -> (x != y?=w3483:bool)
            n2402 = Increment(x=w3479) -> (x+1=w3488:dbl)
            n2403 = case shown="True" w3483 {
              tunnel: w3482 -> [_ w3489]
              frame False {
              }
              frame True {
                n2404 = call "IMAQ AVI Close"("Avi Refnum"=w3489) -> ()  [unwired: 1 in, 10 out]
              }
            }
            n2405 = local write "Video Index"(w3488) -> ()
            n2406 = call "IMAQ AVI Create"("Frames Per Second"=u32 30, "AVI Path"=w3478) -> ("Avi Refnum"=w3486:T39)  [unwired: 5 in, 4 out]
          }
        }
        n2407 = Equal To 0?(x=w3469) -> (x = 0?=w3468:bool)
        n2408 = Select(t=w3459, s=w3460, f=w3457) -> (s? t:f=w3458:T39)
        n2409 = feedback-in #1(w3458) -> ()
        n2410 = case shown="True" w3468 {
          tunnel: w3467 -> [w3490 w3517]
          tunnel: w3466 -> [_ w3516]
          tunnel: [w3490 w3513] -> w3464
          tunnel: w3463 -> [_ w3494]
          tunnel: w3452 -> [_ w3501]
          tunnel: w3458 -> [_ w3499]
          tunnel: w3450 -> [_ w3495]
          tunnel: w3449 -> [_ w3496]
          frame False {
          }
          frame True {
            w3507 = u32 0 ("X-offset IN")
            n2411 = call "DMR_GetImageRequestBufferData.vi"("driver handle IN"=w3517, "request number IN"=w3516) -> ("width OUT"=w3506:i32, "height OUT"=w3505:i32, "driver handle OUT"=w3512:i32, "request number OUT"=w3511:i32, "bytes per pixel OUT"=w3508:i32)  [unwired: 13 out]
            n2412 = call "DMR_GetImageRequestBufferImageData.vi"("driver handle IN"=w3512, "request number IN"=w3511, "bytes per pixel IN"=w3508, "X-offset IN"=w3507, "Y-offset IN"=w3507, "height IN"=w3505, "width IN"=w3506) -> ("driver handle OUT"=w3510:u32, "request number OUT"=w3509:u32, "image OUT"=w3502:u32[][])  [unwired: 10 out]
            n2413 = call "DMR_ImageRequestUnlock.vi"("request number IN"=w3509, "driver handle IN"=w3510) -> ("driver handle OUT"=w3515:i32)  [unwired: 1 in, 2 out]
            n2414 = case shown="True" "Averaging" {
              tunnel: w3502 -> [w3558 w3563]
              tunnel: [w3558 w3562] -> w3498
              tunnel: w3501 -> [_ w3560]
              frame False {
              }
              frame True {
                (unwired) 1
                w3568 = 1
                n2415 = feedback #2(w3560) -> (w3559:u32[][])
                n2416 = Add(x=w3563, y=w3559) -> (x+y=w3564:u32[][])
                n2417 = Select(t=w3560, s="Reset Averaging", f=w3564) -> (s? t:f=w3566:u32[][])
                n2418 = feedback-in #2(w3566) -> ()
                n2419 = feedback #3(w3568) -> (w3561:i32)
                n2420 = Divide(x=w3564, y=w3561) -> (x/y=w3565:dbl[][])
                n2421 = Increment(x=w3561) -> (x+1=w3569:i32)
                n2422 = To Unsigned Long Integer(number=w3565) -> (unsigned 32bit integer=w3562:u32[][])
                n2423 = Select(t=w3568, s="Reset Averaging", f=w3569) -> (s? t:f=w3567:i32)
                n2424 = feedback-in #3(w3567) -> ()
              }
            }
            n2425 = call "DMR_ImageRequestSingle.vi"("request control IN"=0, "driver handle IN"=w3515) -> ("driver handle OUT"=w3513:i32)  [unwired: 3 out]
            n2426 = disable-structure shown="Disabled" {
              disable-tunnel: w3498 -> [w3535 _]
              disable-tunnel: w3495 -> [w3534 _]
              frame Disabled {
                n2427 = To Double Precision Float(number=w3535) -> (double precision float=w3533:dbl[][])
                n2428 = In Range and Coerce(upper limit="Intensity Upper", x=w3533, lower limit="Intensity Lower") -> (coerced(x)=w3532:dbl[][])  [unwired: 1 out]
                n2429 = Subtract(x="Intensity Upper", y="Intensity Lower") -> (x-y=w3529:dbl)
                n2430 = Subtract(x=w3532, y="Intensity Lower") -> (x-y=w3530:dbl[][])
                n2431 = Divide(x=w3530, y=w3529) -> (x/y=w3531:dbl[][])
                n2432 = Multiply(x=255.0, y=w3531) -> (x*y=w3527:dbl[][])
                n2433 = To Unsigned Byte Integer(number=w3527) -> (unsigned 8bit integer=w3536:u8[][])
                n2434 = call "IMAQ ArrayToImage"("Image Pixels (U8)"=w3536, "Image"=w3534) -> ("Image Out"=w3523:T2)  [unwired: 4 in, 5 out]
                n2435 = First Call?() -> (First Call?: T/F=w3524:bool)
                n2436 = case shown="True" w3524 {
                  tunnel: w3523 -> [w3537 w3548]
                  frame False {
                    n2437 = flat-sequence {
                      tunnel: w3537 -> [w3543]
                      frame #0 {
                        w3540 = FALSE ("Get/Set Status? (Set)")
                        w3539 = 0 ("Window Number (0...15)")
                        n2438 = call "IMAQ WindSize"("Get/Set Status? (Set)"=w3540, "Window Number"=w3539) -> ("Width & Height out"=→"Window Size":cluster{"Width":i32, "Height":i32})  [unwired: 4 in, 2 out]
                        n2439 = call "IMAQ WindMove"("Window Number (0...15)"=w3539, "Get/Set Status? (Set)"=w3540) -> ("Coordinates (screen)"=→"Window Position":cluster{"X Position":i32, "Y Position":i32})  [unwired: 3 in, 1 out]
                        n2440 = call "IMAQ WindDraw"("Resize to Image Size? (Y)"=FALSE, "Window Number (0...15)"=w3539, "Image"=w3543) -> ()  [unwired: 7 in, 2 out]
                      }
                      frame #1 {
                        n2441 = call "IMAQ WindZoom 2"("Center Point"="Center Point", "Zoom to Fit? (False)"=FALSE, "Zoom Factor"="Zoom Factor") -> ()  [unwired: 5 in, 4 out]
                      }
                    }
                  }
                  frame True {
                    n2442 = flat-sequence {
                      tunnel: w3548 -> [w3551]
                      tunnel: [w3549] -> w3547
                      tunnel: w3547 -> [w3553]
                      frame #0 {
                        w3550 = TRUE ("Resize to Image Size? (Y)")
                        w3549 = 0 ("Window Number (0...15)")
                        n2443 = call "IMAQ WindNonTearing"("Window Number"=w3549, "NonTearing? (True)"=w3550) -> ()  [unwired: 8 in, 2 out]
                        n2444 = call "IMAQ WindDraw"("Resize to Image Size? (Y)"=w3550, "Window Number (0...15)"=w3549, "Image"=w3551) -> ()  [unwired: 7 in, 2 out]
                      }
                      frame #1 {
                        n2445 = call "IMAQ WindSize"("Scrollbars? (N)"=FALSE, "Width & Height"="Initial Window Size", "Window Number"=w3553) -> ()  [unwired: 3 in, 3 out]
                        n2446 = call "IMAQ WindMove"("Window Number (0...15)"=w3553, "Coordinates (screen)"="Initial Window Position") -> ()  [unwired: 3 in, 2 out]
                      }
                    }
                  }
                }
              }
              frame Enabled {
              }
            }
            n2447 = To Unsigned Byte Integer(number=w3498) -> (unsigned 8bit integer=w3497:u8[][])
            n2448 = call "IMAQ ArrayToImage"("Image Pixels (U8)"=w3497, "Image"=w3494) -> ("Image Out"=w3492:T2)  [unwired: 4 in, 5 out]
            n2449 = case shown="True" "Save Video" {
              tunnel: w3499 -> [_ w3557]
              tunnel: w3492 -> [_ w3556]
              frame False {
              }
              frame True {
                n2450 = call "IMAQ AVI Write Frame"("Image"=w3556, "Avi Refnum"=w3557) -> ()  [unwired: 2 in, 8 out]
              }
            }
            n2451 = case shown="True" "Save Image" {
              tunnel: w3497 -> [_ w3572]
              tunnel: w3496 -> [_ w3571]
              frame False {
              }
              frame True {
                n2452 = call <vilib>:"Flatten Pixmap.vi"("colors"=w3571, "8-bit pixmap"=w3572) -> ("image data"=w3578:T40)  [unwired: 4 in, 5 out]
                n2453 = call "Create new save file.vi"("Insert"="video_frame_" ("string"), "Ext"=".bmp" ("string"), "Index In"="Image Index") -> ("Path Out"=w3574:path, "Index Out"=w3579:dbl)
                n2454 = Increment(x=w3579) -> (x+1=w3573:dbl)
                n2455 = local write "Image Index"(w3573) -> ()
                n2456 = call <vilib>:"Write BMP File.vi"("image data"=w3578, "path to BMP file"=w3574) -> ()  [unwired: 1 in, 9 out]
              }
            }
            n2457 = case shown="True" "Target" {
              tunnel: w3492 -> [w3518 w3522]
              tunnel: [w3518 w3520] -> w3491
              frame False {
              }
              frame True {
                n2458 = local read "Target coordinates"() -> (w3519:cluster{"X1":dbl, "Y1":dbl, "X2":dbl, "Y2":dbl})
                n2459 = call "IMAQ Overlay Oval"("Color"=u32 16711680, "Bounding Rectangle"=w3519, "Image"=w3522) -> ("Image Out"=w3520:T2)  [unwired: 7 in, 1 out]
              }
            }
            "Primary Video Display" <- w3491
          }
        }
        n2460 = node-c288(w3453) -> ()  [unwired: 1 out]
      }
      n2461 = node-c288(w3437) -> ()  [unwired: 1 out]
      n2462 = call "DMR_CloseDevice2.vi"("driver handle IN"=w3442) -> ()  [unwired: 1 in, 4 out]
    }
    frame #4 {
      n2463 = call "DMR_Close.vi"() -> ()  [unwired: 1 out]
    }
  }
  n2464 = local write "Offset (nm)"(0.0 ("Offset (nm)")) -> ()
  n2465 = local write "Bead Mean (nm)"(0.0 ("Bead Mean (nm)")) -> ()
  n2466 = local write "Total Volume\nFlowed P1 (uL)"(w45) -> ()
  n2467 = local write "Total Volume\nFlowed Samp (uL)"(w45) -> ()
  n2468 = local write "Total Volume\nFlowed P3 (uL)"(w45) -> ()
  n2469 = node-c288(i64 1 ("Period"), 1 ("Processor")) -> (w217:T26)  [unwired: 2 out]
  n2470 = timed-loop "Acquire Data" {
    tunnel: w51 -> [w3886]
    tunnel: w98 -> [w3885]
    tunnel: [w3915] -> w309
    tunnel: [w3910] -> w307
    timing: w217 -> [_]
    timing-out: [_] -> w216
    tunnel: w116 -> [w3742]
    stop <- "Stop All" stop-if-true
    w3666 = "Initialize"
    w3732 = "NI_ChannelName" ("name")
    # "I think that the conversion\nfrom 'wiggle amp' to nm\nis 0.277 nm/input. So, 1000\nfor an input is 277 nm."
    n2471 = node-c288() -> ()  [unwired: 2 out]
    n2472 = First Call?() -> (First Call?: T/F=w3701:bool)
    n2473 = Or(x="Reset", y=w3701) -> (x .or. y?=w3702:bool)
    n2474 = local read "Flushing P1"() -> (w3621:bool)
    n2475 = case "Reset data stream" shown="True" w3702 {
      tunnel: w3886 -> [w4951 w4959]
      tunnel: w3885 -> [w4950 w4958]
      tunnel: [w4951 w4953] -> w3614
      tunnel: [w4950 w4952] -> w3881
      frame False {
      }
      frame True {
        w4956 = TRUE ("AI to FIFO")
        n2476 = local write "Overflow (data lost)"(FALSE ("Overflow (data lost)")) -> ()
        n2477 = call "reset FPGA DMA.vi"("error in"=w4958, "FPGA VI Reference In"=w4959) -> ("error out"=w4954:errorcluster, "FPGA VI Reference Out"=w4955:T22)
        n2478 = xnode "Read/Write Control"("FPGA VI Reference In"=w4955, "error in"=w4954, "AI to FIFO"=w4956, "APD to FIFO"=w4956) -> ("FPGA VI Reference Out"=w4953:T22, "error out"=w4952:errorcluster)
      }
    }
    n2479 = case shown="True" w3621 {
      frame False {
      }
      frame True {
        n2480 = local read "Flush rate (uL/m) P1"() -> (w3986:dbl)
        n2481 = local read "HP1 Flush Time (s)"() -> (w3992:dbl)
        n2482 = local read "DMA Update Period (s)"() -> (w3979:dbl)
        n2483 = Divide(x=w3986, y=60.0) -> (x/y=w3978:dbl)
        n2484 = feedback #4(0.0) -> (w3981:dbl)
        n2485 = Divide(x=w3992, y=w3979) -> (x/y=w3984:dbl)
        n2486 = feedback #5(0) -> (w3990:i32)
        n2487 = Increment(x=w3990) -> (x+1=w3983:i32)
        n2488 = Multiply(x=w3979, y=w3978) -> (x*y=w3977:dbl)
        n2489 = Greater?(x=w3983, y=w3984) -> (0:w3989:bool)
        n2490 = Compound Arithmetic op=MULTIPLY(w3979, w3983, w3978) -> (→"P1 Flush Volume (uL)":dbl)
        n2491 = Divide(x=w3983, y=w3984) -> (x/y=→"P1 Flushing Bar":dbl)
        n2492 = Add(x=w3977, y=w3981) -> (x+y=w3980:dbl)
        "Total Volume\nFlowed P1 (uL)" <- w3980
        n2493 = feedback-in #4(w3980) -> ()
        n2494 = case shown="True" w3989 {
          tunnel: w3983 -> [w3993 _]
          tunnel: [w3993 0] -> w3988
          frame False {
          }
          frame True {
            w3994 = FALSE ("Flushing P1")
            n2495 = local write "Inject Pump 1"(w3994) -> ()
            n2496 = local write "Flushing P1"(w3994) -> ()
            n2497 = property on="Clear Volume P1" class="Bool (strict)"("Val(Sgnl)"=TRUE ("Value (Signaling)")) -> ()  [unwired: 2 in, 2 out]
          }
        }
        n2498 = feedback-in #5(w3988) -> ()
      }
    }
    n2499 = Or(x="Start AOD Scan", y="Trap Raster Scan") -> (x .or. y?=w3840:bool)
    n2500 = case "Start AOM raster scan" shown="True" w3840 {
      tunnel: w3614 -> [w4801 w4811]
      tunnel: w3881 -> [w4800 w4810]
      tunnel: [w4801 w4804] -> w3606
      tunnel: [w4800 w4803] -> w3880
      frame False {
      }
      frame True {
        n2501 = case shown="True" "Restart DMA? (AOD)" {
          tunnel: [w4849 w4851] -> w4805
          tunnel: [w4848 w4850] -> w4806
          tunnel: w4811 -> [w4849 w4853]
          tunnel: w4810 -> [w4848 w4852]
          frame False {
          }
          frame True {
            n2502 = local write "Overflow (data lost)"(FALSE ("Overflow (data lost)")) -> ()
            n2503 = call "reset FPGA DMA.vi"("error in"=w4852, "FPGA VI Reference In"=w4853) -> ("error out"=w4850:errorcluster, "FPGA VI Reference Out"=w4851:T22)
          }
        }
        n2504 = local write "Trap Raster Scan"(FALSE ("Trap Raster Scan")) -> ()
        n2505 = case shown="False" "Move MCL Also?" {
          tunnel: w4806 -> [w4815 w4843]
          tunnel: w4805 -> [w4816 w4844]
          tunnel: [w4814 w4847] -> w4804
          tunnel: [w4813 w4846] -> w4803
          frame False {
            w4812 = TRUE ("AI to FIFO")
            n2506 = xnode "Read/Write Control"("FPGA VI Reference In"=w4816, "error in"=w4815, "AI to FIFO"=w4812, "APD to FIFO"=w4812, "Start scan"=w4812) -> ("FPGA VI Reference Out"=w4814:T22, "error out"=w4813:errorcluster)
          }
          frame True {
            w4840 = FALSE ("1D or 2D Scan?")
            w4845 = TRUE ("AI to FIFO")
            # "Count for MCL loop"
            # "N total cycles"
            # "N steps"
            # "V_int"
            n2507 = local read "Scan Range (nm)"() -> (w4822:dbl)